vi "StarlyteSolarSimulator.vi"() -> ()   [LabVIEW 2013]
doc: "# STARLYTE SOLAR SIMULATOR\n# SUBMITTED FOR 2017 NASA INTERNATIONAL SPACE APPS CHALLENGE\n# PROJECT: STARLYTE\n# AUTHORS: ANDREW DENIO\n# DATE: 5/5/2017"
uses:
  <vilib>/Instr/_visa.llb/VISA Configure Serial Port (Instr).vi
  <vilib>/regexp/Match Regular Expression.xnode
panel:
  out "substring":string
  out "Heading":dbl
  out "Heading":string
  out "x = y?":bool
  out "Tilt":string
  out "Tilt Angle":dbl
  out "Effeciency Percentage":dbl
  in  "Watts Per HI-SEAs Panel":dbl=280.0 format="%#_13g"
  in  "Watts per SunnyTech Panel":dbl=1.25 format="%#_13g"
  in  "Number of Panels in Array":dbl=36.0 format="%#_13g"
  in  "stop":bool
  out "Current":string
  out "Voltage":string
  out "String from Arduino":string
  in  "COMM for Solar Panel":refnum<visa-resource-name>="COM12"
  out "# of SunnyTech Panels":dbl
  out "# of SunnyTech Panels":dbl
  out "Simulated Power (W)":dbl
  out "Simulated Current (A)":dbl
  out "Simulated Voltage (V)":dbl
  out "Raw Power (W)":dbl
  out "Raw Current (A)":dbl
  out "Raw Voltage (V)":dbl
  out "Gauge 3":dbl(knob)=3.421631877688583 scale=0.0..30.0
  out "Battery Charge (kWh)":dbl(slide) scale=0.0..100.0
  in  "Dial":dbl(knob) scale=0.0..10.0
  out "Array Power (W)":dbl
  out "Array Current (A)":dbl
  out "Array Voltage (V)":dbl
  out "Gauge":dbl(knob) scale=0.0..20500.0
  in  "# SunnyTech Panels to Simulate:":dbl=1.0
  in  "\"Sun\" Input Wattage:":dbl=60.0
  # "solar simulator"
  # "SunnyTech Panel:"
  # "HI-SEAs Array:"
  # "HI-SEAs Panel:"
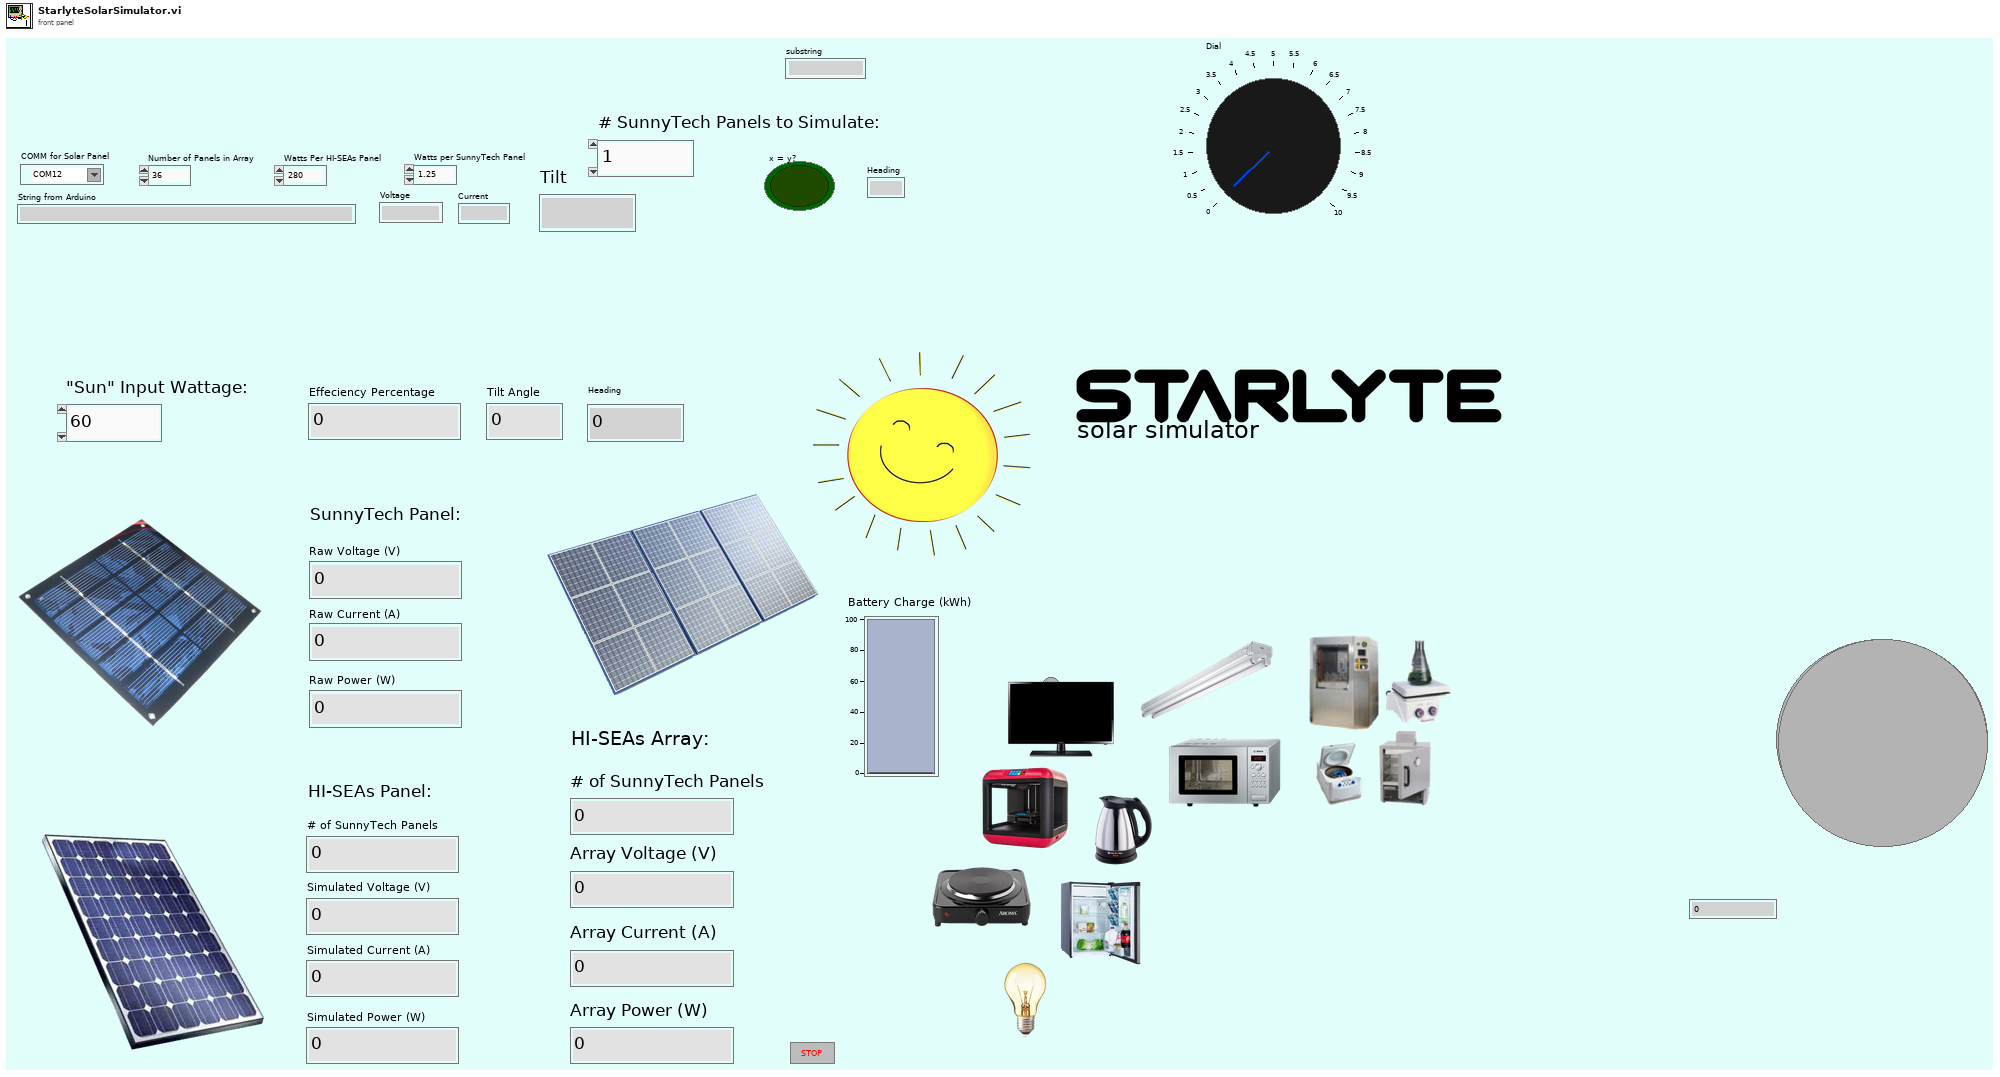
[diagram p1: front panel]
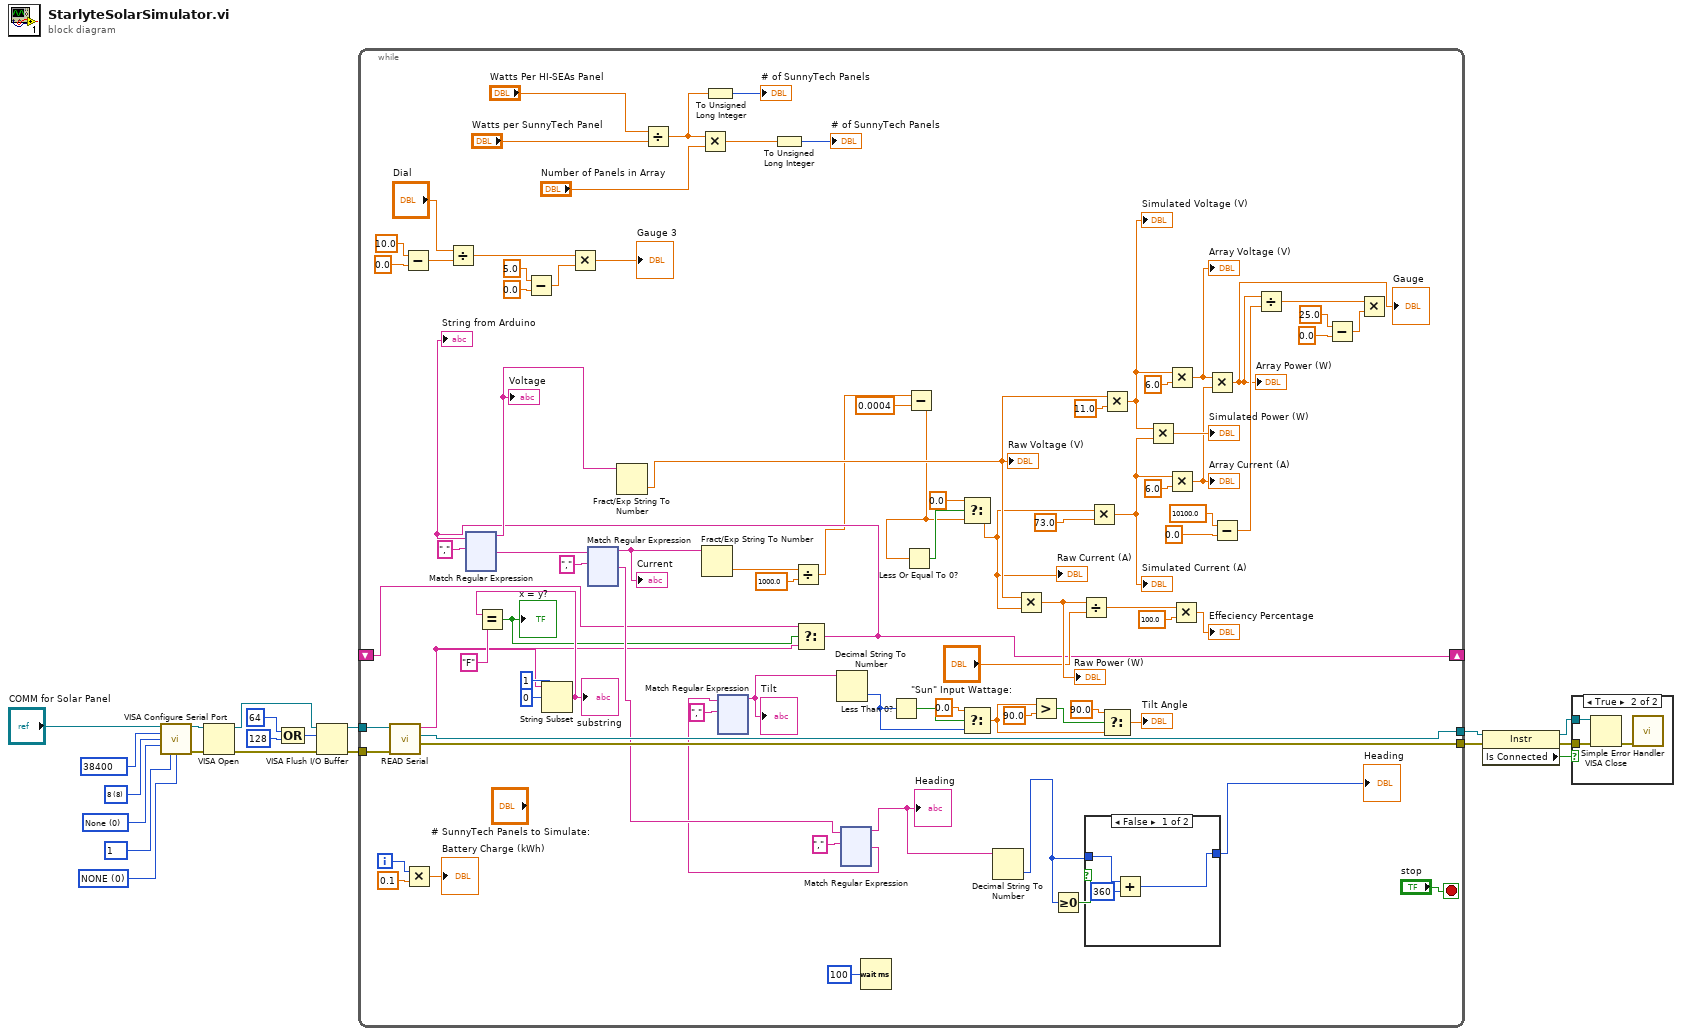
[diagram p0: block diagram]
diagram:
  w14 = u16 0 items=["NONE", "XON/XOFF", "RTS/CTS", "XON/XOFF & RTS/CTS", "DTR/DSR", "XON/XOFF & DTR/DSR"] ("flow control")
  w15 = u16 10 items=["1"=10, "1.5"=15, "2"=20] ("stop bits")
  w16 = u16 0 items=["None", "Odd", "Even", "Mark", "Space"] ("parity")
  w17 = u16 8 items=["8"=8, "7"=7, "6"=6, "5"=5] ("data bits")
  w8 = u32 38400 items=["1200"=1200, "2400"=2400, "4800"=4800, "9600"=9600, "19200"=19200, "38400"=38400, "57600"=57600, "115200"=115200] ("baud rate")
  n1 = call-poly "VISA Configure Serial Port"("VISA resource name"="COMM for Solar Panel", "baud rate (9600)"=w8, "data bits (8)"=w17, "parity (0:none)"=w16, "stop bits (10: 1 bit)"=w15, "flow control (0:none)"=w14) -> ("VISA resource name out"=w20:refnum<visa-resource-name>, "error out"=w19:errorcluster)  [unwired: 1 in, 7 out]
  n2 = VISA Open(error in (no error)=w19, VISA resource name=w20) -> (VISA resource name=w13:refnum<visa-resource-name>, error out=w9:errorcluster)  [unwired: 3 out]
  n3 = Compound Arithmetic op=OR(64, 128) -> (w10:i32)
  n4 = VISA Flush I/O Buffer(VISA resource name=w13, mask (16)=w10, error in (no error)=w9) -> (VISA resource name out=w7:refnum<visa-resource-name>, error out=w6:errorcluster)
  n5 = while {
    tunnel: w7 -> [w106]
    tunnel: w6 -> [w105]
    tunnel: [w104] -> w2
    tunnel: [w103] -> w1
    shift-right: [w31] -> _
    shift-left: _ -> [w32]
    i -> [w87]
    stop <- "stop" stop-if-true
    n6 = call "READ Serial.vi"("error in"=w105, "VISA Resource Name In"=w106) -> ("error out"=w103:errorcluster, "VISA Resource Name Out"=w104:refnum<visa-resource-name>, "Output String"=w33:string)  [unwired: 4 in]
    n7 = Subtract(x=10.0, y=0.0) -> (x-y=w96:dbl)
    n8 = Multiply(x=w87, y=0.1) -> (x*y=→"Battery Charge (kWh)":dbl)
    n9 = Divide(x="Dial", y=w96) -> (x/y=w97:dbl)
    n10 = Subtract(x=5.0, y=0.0) -> (x-y=w94:dbl)
    n11 = String Subset(string=w33, offset (0)=0, length (rest)=1 ("length (rest)")) -> (substring=w35:string)
    "substring" <- w35
    n12 = Equal?(x=w35, y="F" ("regular expression")) -> (x = y?=w34:bool)
    "x = y?" <- w34
    n13 = Multiply(x=w97, y=w94) -> (x*y=→"Gauge 3":dbl)
    n14 = Divide(x="Watts Per HI-SEAs Panel", y="Watts per SunnyTech Panel") -> (x/y=w80:dbl)
    n15 = Multiply(x=w80, y="Number of Panels in Array") -> (x*y=w78:dbl)
    n16 = To Unsigned Long Integer(number=w80) -> (unsigned 32bit integer=→"# of SunnyTech Panels":u32)
    n17 = To Unsigned Long Integer(number=w78) -> (unsigned 32bit integer=→"# of SunnyTech Panels":u32)
    n18 = Select(t=w32, s=w34, f=w33) -> (s? t:f=w31:string)
    "String from Arduino" <- w31
    n19 = xnode "Match Regular Expression"("input string"=w31, "regular expression"=",") -> ("before match"=w45:string, "after match"=w100:string)  [unwired: 2 in, 5 out]
    "Voltage" <- w45
    n20 = xnode "Match Regular Expression"("input string"=w100, "regular expression"=",") -> ("before match"=w48:string, "after match"=w40:string)  [unwired: 2 in, 5 out]
    "Current" <- w48
    n21 = Fract/Exp String To Number(string=w45) -> (number=w44:dbl)  [unwired: 3 in, 1 out]
    "Raw Voltage (V)" <- w44
    n22 = Fract/Exp String To Number(string=w48) -> (number=w47:dbl)  [unwired: 3 in, 1 out]
    n23 = Divide(x=w47, y=1000.0) -> (x/y=w24:dbl)
    n24 = xnode "Match Regular Expression"("input string"=w40, "regular expression"=",") -> ("before match"=w39:string, "after match"=w38:string)  [unwired: 2 in, 5 out]
    "Heading" <- w39
    n25 = xnode "Match Regular Expression"("input string"=w38, "regular expression"=",") -> ("before match"=w57:string)  [unwired: 2 in, 6 out]
    "Tilt" <- w57
    n26 = Decimal String To Number(string=w57) -> (number=w54:i32)  [unwired: 2 in, 1 out]
    n27 = Wait (ms)(milliseconds to wait=u32 100) -> ()  [unwired: 1 out]
    n28 = Less Than 0?(x=w54) -> (x < 0?=w56:bool)
    n29 = Subtract(x=w24, y=0.0004) -> (x-y=w22:dbl)
    n30 = Less Or Equal To 0?(x=w22) -> (x <= 0?=w25:bool)
    n31 = Select(t=0.0, s=w25, f=w22) -> (s? t:f=w29:dbl)
    "Raw Current (A)" <- w29
    n32 = Select(t=0.0, s=w56, f=w54) -> (s? t:f=w50:dbl)
    n33 = Decimal String To Number(string=w39) -> (number=w27:i32)  [unwired: 2 in, 1 out]
    n34 = Multiply(x=w44, y=w29) -> (x*y=w60:dbl)
    "Raw Power (W)" <- w60
    n35 = Greater?(x=w50, y=90.0) -> (0:w52:bool)
    n36 = Greater Or Equal To 0?(x=w27) -> (x >= 0?=w28:bool)
    n37 = Divide(x=w60, y="\"Sun\" Input Wattage:") -> (x/y=w61:dbl)
    n38 = case shown="False" w28 {
      tunnel: w27 -> [w109 w110]
      tunnel: [w107 w110] -> w26
      frame False {
        n39 = Add(x=w109, y=360) -> (x+y=w107:i32)
      }
      frame True {
      }
    }
    "Heading" <- w26
    n40 = Multiply(x=w29, y=73.0) -> (x*y=w81:dbl)
    "Simulated Current (A)" <- w81
    n41 = Multiply(x=w44, y=11.0) -> (x*y=w75:dbl)
    "Simulated Voltage (V)" <- w75
    n42 = Select(t=90.0, s=w52, f=w50) -> (s? t:f=→"Tilt Angle":dbl)
    n43 = Multiply(x=w75, y=w81) -> (x*y=→"Simulated Power (W)":dbl)
    n44 = Multiply(x=w75, y=6.0) -> (x*y=w73:dbl)
    "Array Voltage (V)" <- w73
    n45 = Multiply(x=w81, y=6.0) -> (x*y=w72:dbl)
    "Array Current (A)" <- w72
    n46 = Multiply(x=w61, y=100.0) -> (x*y=→"Effeciency Percentage":dbl)
    n47 = Multiply(x=w73, y=w72) -> (x*y=w43:dbl)
    "Gauge" <- w43
    "Array Power (W)" <- w43
    n48 = Subtract(x=10100.0, y=0.0) -> (x-y=w65:dbl)
    n49 = Divide(x=w43, y=w65) -> (x/y=w64:dbl)
    n50 = Subtract(x=25.0, y=0.0) -> (x-y=w66:dbl)
    n51 = Multiply(x=w64, y=w66) -> ()  [unwired: 1 out]
  }
  n52 = property class="Instr"(reference=w2, error in=w1) -> (reference out=w3:refnum<visa-resource-name>, error out=w4:errorcluster, "Is Connected"=w5:bool)
  n53 = case shown="True" w5 {
    tunnel: w3 -> [_ w569]
    tunnel: w4 -> [_ w568]
    frame False {
    }
    frame True {
      n54 = VISA Close(VISA resource name=w569, error in (no error)=w568) -> (error out=w567:errorcluster)
      n55 = call <vilib>:"Simple Error Handler.vi"("error in (no error)"=w567) -> ()  [unwired: 1 in, 8 out]
    }
  }
